vi "MPS_Mag_Core.vi"(0 "EmptyBoreBaseline_Mag_BMon":dbl[](array[numeric])=array[420000 elements], 5 "EmptyBoreBaseline_Mag":dbl[](array[numeric])=array[420000 elements]) -> (1 "Samples Per Acquisition":dbl=21000.0, 3 "Drive IMon":waveform(dbl), 4 "Susceptibility Curves":cluster{"Y":dbl[], "Y":dbl[]}[](graph), 6 "Rx Smooth":dbl[](graph), 10 "BMon_Smooth":dbl[](graph), 12 "Bias Current":waveform(dbl)(graph)={"t0"=timestamp(3727906504.0247726 s since 1904-01-01), "dt"=9.9999999999997e-07, "Y"=array[420000 elements], "attributes"=variant("NI_ChannelName"=variant(string "H1/ai5"), "NI_UnitDescription"=variant(string "Volts"))}, 13 "Rx_Raw":waveform(dbl), 14 "RxBaselineSub":waveform(dbl)(graph), 15 "Bias Smooth":dbl[](graph))   [LabVIEW 2021]
uses:
  <extravilib>/ChannelInstances/Tag-dbl/Write With Abort.vi
  MPS_global_variables.vi
  <extravilib>/ChannelInstances/Tag-dbl/Instantiate.vi
  <extravilib>/ChannelInstances/Tag-dbl/Endpoint.vi
  <extravilib>/ChannelInstances/Tag-dbl.lvlib
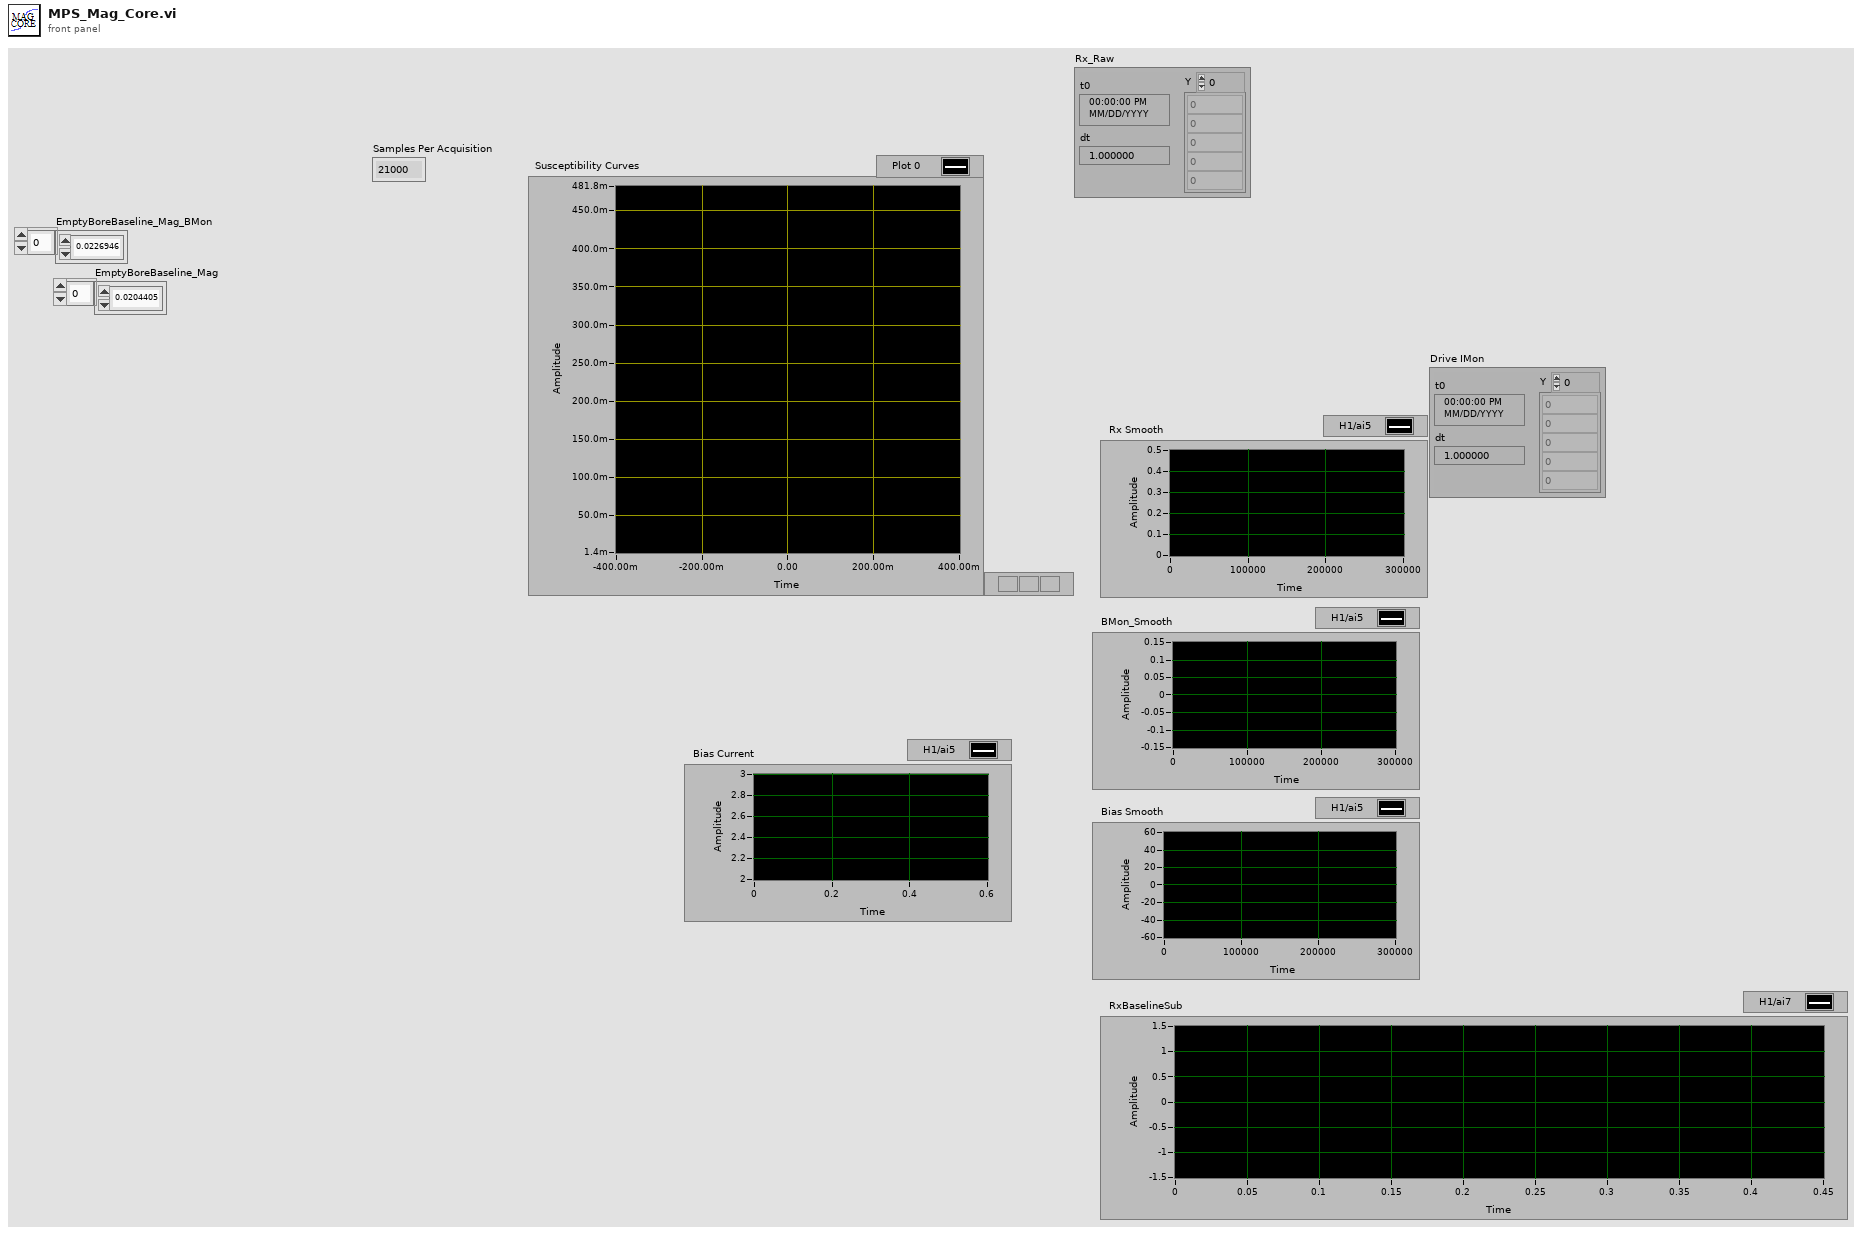
[diagram p1: front panel]
types:
  T1 = typedef "Tag-dbl.lvlib/))Channel.ctl" = refnum<queue>
  T2 = cluster{"sample rate":dbl, "Tx freq":dbl, "Tx amp":dbl, "Tx cycles\nSpectroscopy":dbl, "Bias amp":dbl, "Bias freq":dbl, "Receive range":dbl, "Bias Periods\nMagnetometry":dbl, "Tx Freq Division Factor":dbl, "Drive Periods per Bias":dbl, "TX harmonics":dbl[]}
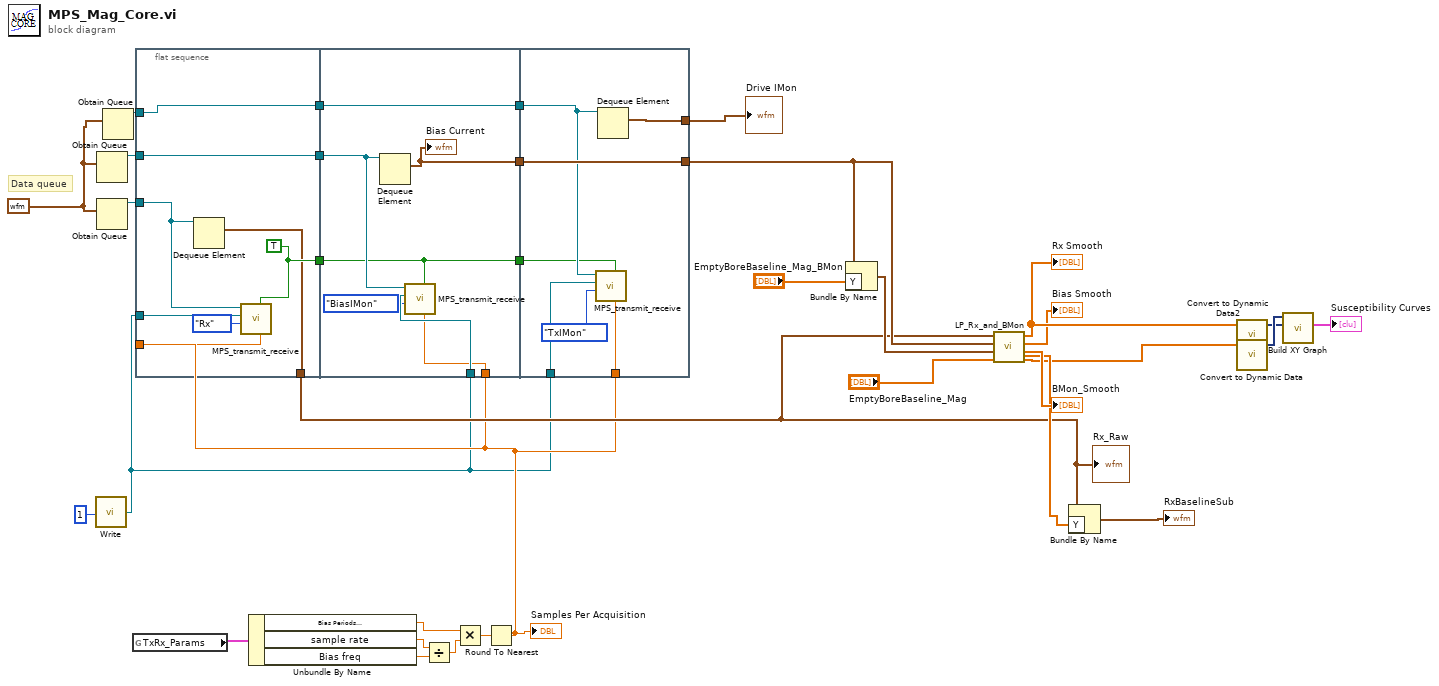
[diagram p0: block diagram]
diagram:
  w9 = waveform(dbl) {"t0"=timestamp(0 s since 1904-01-01), "dt"=1.0, "Y"=[]} ("Waveform")
  # "Data queue"
  n1 = call <extravilib>:"Write.vi"("element"=1 ("number of readouts")) -> ("channel"=w3:T1)  [unwired: 1 out]
  n2 = Obtain Queue(element data type=w9) -> (queue out=w30:refnum<queue>)  [unwired: 4 in, 2 out]
  n3 = Obtain Queue(element data type=w9) -> (queue out=w31:refnum<queue>)  [unwired: 4 in, 2 out]
  n4 = Obtain Queue(element data type=w9) -> (queue out=w6:refnum<queue>)  [unwired: 4 in, 2 out]
  n5 = global read "MPS_global_variables.vi" "TxRx_Params"() -> (w24:T2)
  n6 = flat-sequence {
    tunnel: w31 -> [w41]
    tunnel: [w40] -> w34
    tunnel: w3 -> [w42]
    tunnel: w30 -> [w40]
    tunnel: [w37] -> w11
    tunnel: w4 -> [w39]
    tunnel: [w38] -> w33
    tunnel: [w36] -> w7
    tunnel: w6 -> [w36]
    tunnel: w34 -> [w49]
    tunnel: w3 -> [w48]
    tunnel: w4 -> [w47]
    tunnel: w33 -> [w43]
    tunnel: [w46] -> w10
    tunnel: [w45] -> w8
    tunnel: w7 -> [w45]
    tunnel: [w43] -> w2
    tunnel: [w56] -> w17
    tunnel: w10 -> [w56]
    tunnel: w8 -> [w54]
    tunnel: [w55] -> w5
    tunnel: w4 -> [w52]
    tunnel: w3 -> [w51]
    tunnel: w2 -> [w50]
    frame #0 {
      w38 = TRUE ("Use Bias? 5")
      n7 = Dequeue Element(queue=w41) -> (element=w37:waveform(dbl))  [unwired: 2 in, 3 out]
      n8 = call "MPS_transmit_receive.vi"("samples per readout"=w39, "Use Bias?"=w38, "InputChans"=enum16{"Rx", "BiasIMon", "TxIMon", "BMon"}."Rx", "channel input for max readouts"=w42, "Measurement Queue"=w41) -> ()  [unwired: 7 in]
    }
    frame #1 {
      n9 = Dequeue Element(queue=w49) -> (element=w46:waveform(dbl))  [unwired: 2 in, 3 out]
      "Bias Current" <- w46
      n10 = call "MPS_transmit_receive.vi"("samples per readout"=w47, "Use Bias?"=w43, "InputChans"=enum16{"Rx", "BiasIMon", "TxIMon", "BMon"}."BiasIMon", "channel input for max readouts"=w48, "Measurement Queue"=w49) -> ()  [unwired: 7 in]
    }
    frame #2 {
      n11 = call "MPS_transmit_receive.vi"("samples per readout"=w52, "Use Bias?"=w50, "InputChans"=enum16{"Rx", "BiasIMon", "TxIMon", "BMon"}."TxIMon", "channel input for max readouts"=w51, "Measurement Queue"=w54) -> ()  [unwired: 7 in]
      n12 = Dequeue Element(queue=w54) -> (element=w55:waveform(dbl))  [unwired: 2 in, 3 out]
    }
  }
  n13 = Unbundle By Name(w24) -> ("Bias Periods\nMagnetometry"=w20:dbl, "sample rate"=w23:dbl, "Bias freq"=w22:dbl)
  n14 = Divide(x=w23, y=w22) -> (x/y=w21:dbl)
  n15 = Multiply(x=w20, y=w21) -> (x*y=w19:dbl)
  n16 = Round To Nearest(number=w19) -> (nearest integer value=w4:dbl)
  "Samples Per Acquisition" <- w4
  n17 = Bundle By Name(cluster=w17, "Y"="EmptyBoreBaseline_Mag_BMon") -> (w16:waveform(dbl))
  n18 = call "LP_Rx_and_BMon.vi"("Rx"=w11, "Bias"=w17, "BMon"=w16, "BaselineSig"="EmptyBoreBaseline_Mag") -> ("RxBaselineSub"=w13:dbl[], "RX_Smooth"=w26:dbl[], "BiasSmooth"=→"Bias Smooth":dbl[], "BMon Smooth"=→"BMon_Smooth":dbl[], "Bias Reconstructed"=w1:dbl[])  [unwired: 1 in]
  "Rx Smooth" <- w26
  n19 = Bundle By Name(cluster=w11, "Y"=w13) -> (→"RxBaselineSub":waveform(dbl))
  n20 = call "Convert to Dynamic Data2"("Array"=w26) -> ("Dynamic Data Type"=w27:dynamicdata)  [unwired: 3 in]
  n21 = call "Convert to Dynamic Data"("Array"=w1) -> ("Dynamic Data Type"=w28:dynamicdata)  [unwired: 3 in]
  n22 = call "Build XY Graph"("Y Input"=w27, "X Input"=w28) -> ("XY Graph"=→"Susceptibility Curves":cluster{"X":dbl[], "Y":dbl[]}[])  [unwired: 8 in, 1 out]
  "Drive IMon" <- w5
  "Rx_Raw" <- w11
